vi "SETI_FPGA Interface v3.vi"() -> ()   [LabVIEW 2015]
uses:
  <vilib>/rvi/interface/RandomDataEmulation/nirviRandomDataOpen.vi
  <vilib>/rvi/interface/common/niFpgaCacheSessionInfoDynamic.vi
  <vilib>/Utility/error.llb/Error Cluster From Error Code.vi
  <vilib>/rvi/errors/niLvFpgaAdjustHostInterfaceError.vi
  <vilib>/rvi/interface/common/niFpgaWaitOnOcc.vi
  <vilib>/FPGAPlugInAG/Dynamic/niLvFpga_Close_Dynamic.vi
  <vilib>/rvi/interface/nirviOpenFPGA/nirviOpenFPGA.xnode
  FPGA Target/Old/SETI_Host_Interface v3.vi
  <vilib>/rvi/interface/nirviReadWriteControl/nirviReadWriteControl.xnode
  <vilib>/rvi/interface/nirviMethod/nirviMethod.xnode
  <vilib>/rvi/interface/nirviCloseFPGA/nirviCloseFPGA.xnode
  <vilib>/rvi/interface/Simulation/niFpgaSimulationCallBeginRW.vi
  <vilib>/rvi/errors/niLvFpgaMergeErrorWithErrorCode.vi
  <vilib>/FPGAPlugInAG/Dynamic/niLvFpga_ReadFifo_Dynamic.vi
  <vilib>/FPGAPlugInAG/Dynamic/niLvFpga_ConfigureFifo_Dynamic.vi
  <vilib>/Analysis/NI_AALBase.lvlib
  NiFpgaLv.dll
  <vilib>/FPGAPlugInAG/Dynamic/niLvFpga_WriteFifo_Dynamic.vi
panel:
  out "Waveform Graph":sgl[][](graph)
  out "Accepted (parsed)":csg[](array[numeric]) format="%_8g"
  in  "index":i32
  in  "Collector Loop":i32=10
  in  "ChirpData accepted":csg[](array[numeric])=array[262144 elements]
  out "Results":csg[](array[numeric]) format="%_8g"
  in  "ChirpData":csg[](array[numeric])=array[262144 elements] format="%_8g"
  out "Chirp/Fft Pair 1 - Chirp Rate 2":fxp<+/-,64,32> format="%.42g"
  in  "Chirp/Fft Pair 1 - Chirp Rate":dbl=0.00554556
  out "State":T1(ring)
  out "%Error":sgl[](array[numeric]) format="%_4e"
  in  "Inputs":i32=2500
  out "Ok?":bool
  out "Start":bool
  out "FPGA Loop Count":i32
  out "Total":u64
  out "Count":u64
  out "Loop Count":i32
  out "Elements Remaining":u32
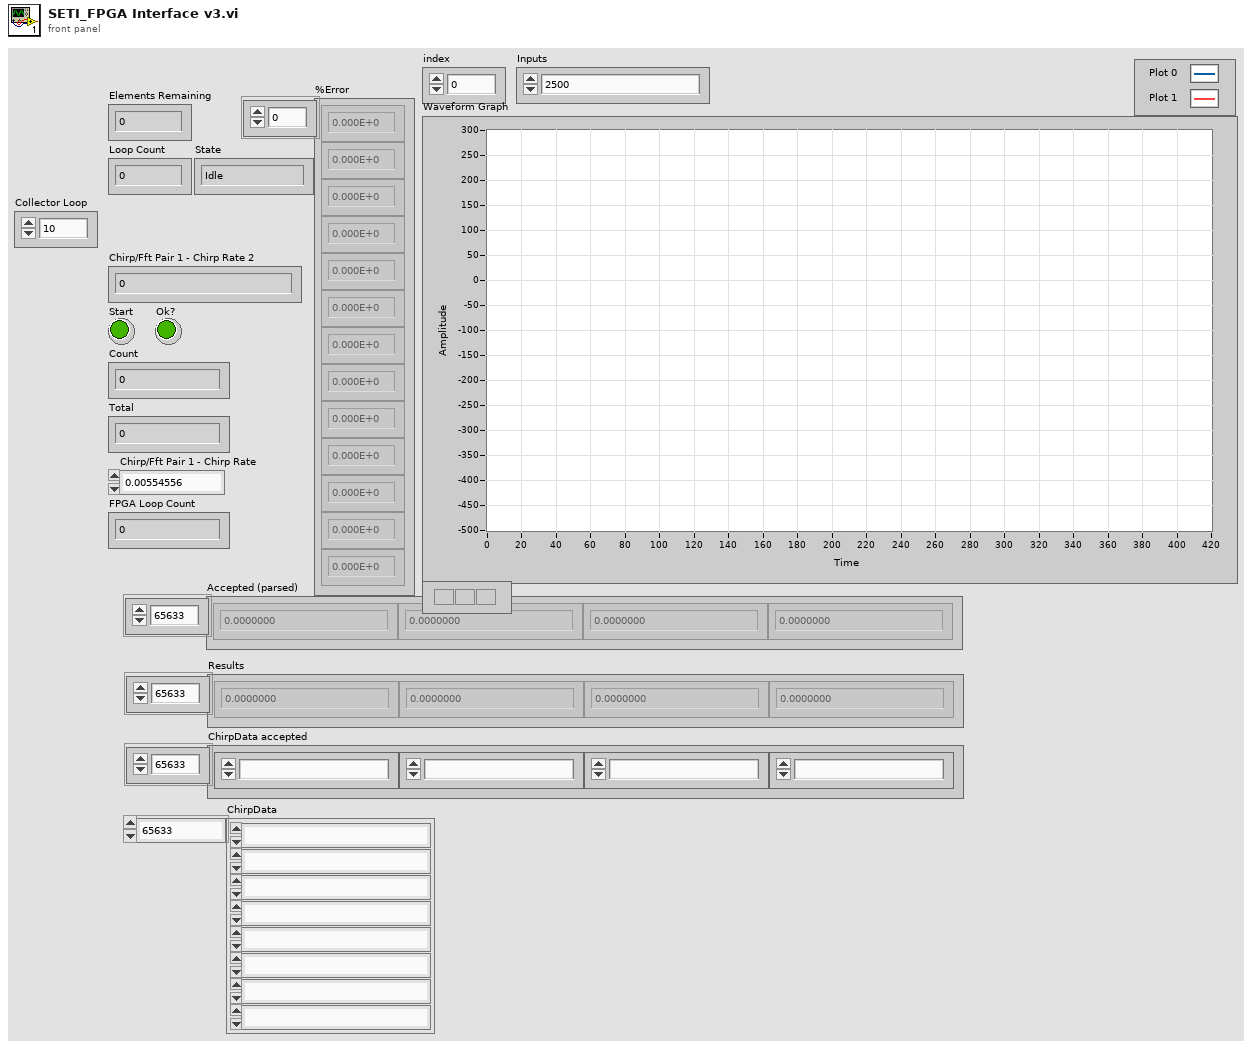
[diagram p1: front panel]
types:
  T1 = enum16{"Idle", "GetNumPoints", "GetChirpRate", "Process", "Stop"}
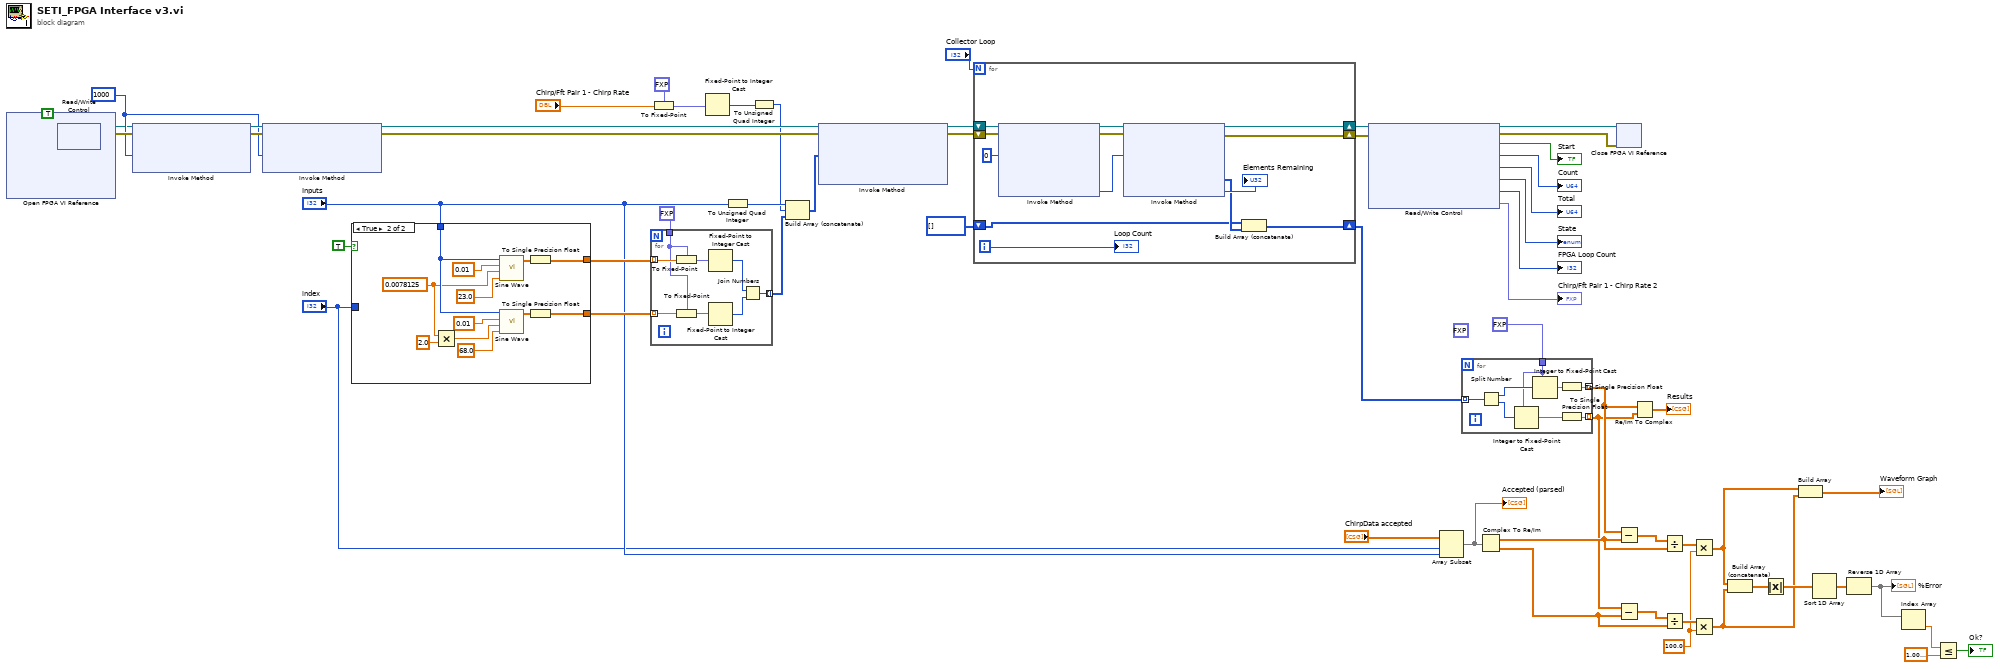
[diagram p0: block diagram]
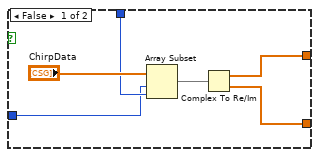
[diagram p2: hidden frame]
diagram:
  (unwired) fxp<+/-,49,4> 0.0 ("Real Out")
  w29 = sgl 100.0
  w45 = u32 1000 ("Requested Depth")
  n1 = xnode "Open FPGA VI Reference"() -> ("FPGA VI Reference Out"=w62:refnum<k20>, "error out"=w61:errorcluster)  [unwired: 2 in]
  n2 = xnode "Read/Write Control"("FPGA VI Reference In"=w62, "error in"=w61, "Start"=TRUE ("Boolean")) -> ("FPGA VI Reference Out"=w41:refnum<k20>, "error out"=w48:errorcluster)
  n3 = xnode "Invoke Method"("FPGA VI Reference In"=w41, "error in"=w48, "Requested Depth"=w45) -> ("FPGA VI Reference Out"=w47:refnum<k20>, "error out"=w46:errorcluster)  [unwired: 1 out]
  n4 = xnode "Invoke Method"("FPGA VI Reference In"=w47, "error in"=w46, "Requested Depth"=w45) -> ("FPGA VI Reference Out"=w44:refnum<k20>, "error out"=w43:errorcluster)  [unwired: 1 out]
  n5 = case shown="True" TRUE {
    tunnel: "Inputs" -> [w64 w74]
    tunnel: [w67 w70] -> w35
    tunnel: [w66 w69] -> w34
    tunnel: "index" -> [w63 _]
    frame False {
      n6 = Array Subset(array="ChirpData", index=w63, length=w64) -> (w65:csg[])
      n7 = Complex To Re/Im(x + iy=w65) -> (x=w67:sgl[], y=w66:sgl[])
    }
    frame True {
      w73 = 0.0078125 ("frequency")
      n8 = Multiply(x=w73, y=2.0) -> (x*y=w71:dbl)
      n9 = call <vilib>:"Sine Wave.vi"("samples"=w74, "amplitude"=0.01, "frequency"=w73, "phase in"=23.0) -> ("sine wave"=w76:dbl[])  [unwired: 1 in, 2 out]
      n10 = call <vilib>:"Sine Wave.vi"("samples"=w74, "amplitude"=0.01, "frequency"=w71, "phase in"=68.0) -> ("sine wave"=w75:dbl[])  [unwired: 1 in, 2 out]
      n11 = To Single Precision Float(number=w76) -> (single precision float=w70:sgl[])
      n12 = To Single Precision Float(number=w75) -> (single precision float=w69:sgl[])
    }
  }
  n13 = for {
    tunnel: w35 -> [w88] mode=indexing
    tunnel: w34 -> [w84] mode=indexing
    tunnel: [w82] -> w36 mode=indexing
    tunnel: fxp<+/-,32,1> 0.0 ("real data in") -> [w81]
    n14 = To Fixed-Point(fixed-point type=w81, number=w88) -> (fixed-point=w87:fxp<+/-,32,1>)
    n15 = To Fixed-Point(fixed-point type=w81, number=w84) -> (fixed-point=w85:fxp<+/-,32,1>)
    n16 = Fixed-Point to Integer Cast(1:w87) -> (0:w86:i32)
    n17 = Fixed-Point to Integer Cast(1:w85) -> (0:w83:i32)
    n18 = Join Numbers(hi=w86, lo=w83) -> ((hi.lo)=w82:u64)
  }
  n19 = To Fixed-Point(fixed-point type=fxp<+/-,64,32> 0.0 ("Chirp/Fft Pair 1 - Chirp Rate"), number="Chirp/Fft Pair 1 - Chirp Rate") -> (fixed-point=w19:fxp<+/-,64,32>)
  n20 = Fixed-Point to Integer Cast(1:w19) -> (0:w18:i64)
  n21 = To Unsigned Quad Integer(1:"Inputs") -> (0:w39:u64)
  n22 = To Unsigned Quad Integer(1:w18) -> (0:w17:u64)
  n23 = Build Array (concatenate)(w39, w17, w36) -> (w40:u64[])
  n24 = xnode "Invoke Method"("FPGA VI Reference In"=w44, "error in"=w43, "Data"=w40) -> ("FPGA VI Reference Out"=w59:refnum<k20>, "error out"=w58:errorcluster)  [unwired: 1 in, 1 out]
  n25 = for {
    N: "Collector Loop" -> [_]
    shift-right: [w89] -> w38
    shift-left: u64[] [] -> [w99]
    shift-right: [w97] -> w55
    shift-left: w59 -> [w95]
    shift-right: [w96] -> w54
    shift-left: w58 -> [w94]
    i -> [w98]
    n26 = xnode "Invoke Method"("FPGA VI Reference In"=w95, "error in"=w94, "Number of Elements"=u32 0) -> ("FPGA VI Reference Out"=w93:refnum<k20>, "error out"=w92:errorcluster, "Elements Remaining"=w90:u32)  [unwired: 1 in, 1 out]
    n27 = xnode "Invoke Method"("FPGA VI Reference In"=w93, "error in"=w92, "Number of Elements"=w90) -> ("FPGA VI Reference Out"=w97:refnum<k20>, "error out"=w96:errorcluster, "Data"=w100:u64[], "Elements Remaining"=→"Elements Remaining":u32)  [unwired: 1 in]
    n28 = Build Array (concatenate)(w99, w100) -> (w89:u64[])
    "Loop Count" <- w98
  }
  n29 = xnode "Read/Write Control"("FPGA VI Reference In"=w55, "error in"=w54) -> ("FPGA VI Reference Out"=w50:refnum<k20>, "error out"=w49:errorcluster, "Start"=→"Start":bool, "Count"=→"Count":u64, "Total"=→"Total":u64, "State"=→"State":T1, "FPGA Loop Count"=→"FPGA Loop Count":i32, "Chirp/Fft Pair 1 - Chirp Rate"=→"Chirp/Fft Pair 1 - Chirp Rate 2":fxp<+/-,64,32>)
  n30 = Array Subset(array="ChirpData accepted", index="index", length="Inputs") -> (w5:csg[])
  "Accepted (parsed)" <- w5
  n31 = for {
    tunnel: w38 -> [w109] mode=indexing
    tunnel: [w108] -> w9 mode=indexing
    tunnel: [w107] -> w8 mode=indexing
    tunnel: fxp<+/-,32,1> 0.0 ("real data in") -> [w104]
    n32 = Split Number(x=w109) -> (hi(x)=w106:u32, lo(x)=w105:u32)
    n33 = Integer to Fixed-Point Cast(fixed-point type=w104, integer=w105) -> (fixed-point=w102:fxp<+/-,32,1>)
    n34 = Integer to Fixed-Point Cast(fixed-point type=w104, integer=w106) -> (fixed-point=w103:fxp<+/-,32,1>)
    n35 = To Single Precision Float(number=w103) -> (single precision float=w108:sgl)
    n36 = To Single Precision Float(number=w102) -> (single precision float=w107:sgl)
  }
  n37 = Complex To Re/Im(x + iy=w5) -> (x=w11:sgl[], y=w10:sgl[])
  n38 = xnode "Close FPGA VI Reference"("FPGA VI Reference In"=w50, "error in"=w49) -> ()  [unwired: 1 out]
  n39 = Subtract(x=w9, y=w11) -> (x-y=w33:sgl[])
  n40 = Subtract(x=w8, y=w10) -> (x-y=w32:sgl[])
  n41 = Re/Im To Complex(1:w8, 2:w9) -> (0:→"Results":csg[])
  n42 = Divide(x=w33, y=w11) -> (x/y=w31:sgl[])
  n43 = Divide(x=w32, y=w10) -> (x/y=w30:sgl[])
  n44 = Multiply(x=w31, y=w29) -> (x*y=w3:sgl[])
  n45 = Multiply(x=w30, y=w29) -> (x*y=w2:sgl[])
  n46 = Build Array (concatenate)(w3, w2) -> (w28:sgl[])
  n47 = Absolute Value(x=w28) -> (abs(x)=w4:sgl[])
  n48 = Build Array(w3, w2) -> (→"Waveform Graph":sgl[][])
  n49 = Sort 1D Array(array=w4) -> (sorted array=w27:sgl[])
  n50 = Reverse 1D Array(array=w27) -> (reversed array=w26:sgl[])
  "%Error" <- w26
  n51 = Index Array(array=w26) -> (element=w25:sgl)  [unwired: 1 in]
  n52 = Less Or Equal?(x=w25, y=sgl 1e-07) -> (x <= y?=→"Ok?":bool)
